vi "UHR-Fleezers Control (host) - 12.3.1.vi"() -> ()   [LabVIEW 2012] (continued)
      tunnel: [_ _ _ _ _ _ _ _ _ w1722 _ _ _ _ _ _ _ _ _ _ _ _ _ _ _ _ _ _ _ _ _ _ _ _ _ _ _ _ _ _ _ _ _ _ _ _ _ _ _ _ _ _ _ _ _ _ _ _ _ _ _ _ _ _ _ _ _ _ _ _ _ _ _ _] -> w1588
      tunnel: [_ _ _ _ _ _ _ "Round T1 X" _ _ _ _ _ _ _ _ _ _ _ _ _ _ _ _ _ _ _ _ _ _ _ _ _ _ _ _ _ _ _ _ _ _ _ _ _ _ _ _ _ _ _ _ _ _ _ _ _ _ _ _ _ _ _ _ _ _ _ _ _ _ _ _ _ _] -> _
      tunnel: [_ _ _ "Adjust Scale\nto Mean" _ _ _ _ _ _ _ _ _ _ _ _ _ _ _ _ _ _ _ _ _ _ _ _ "Test ttrig" _ _ _ _ _ _ _ _ _ _ _ _ _ _ _ _ _ _ "Flush Sample" "Flush Pump 3" "Flush Pump 1" "Clear Volume" _ _ _ _ _ _ _ _ _ _ _ _ _ _ _ _ _ _ _ _ _ _ _] -> _
      tunnel: [_ _ _ _ _ _ _ _ "Round T2 X" _ "Delayed Interlace Start" _ _ _ _ _ _ _ _ _ _ _ _ _ _ _ _ _ _ _ _ _ _ _ _ _ _ _ _ _ _ _ _ _ _ _ _ _ _ _ _ _ _ _ _ _ _ _ _ _ _ _ _ _ _ _ _ _ _ _ _ _ _ _] -> _
      tunnel: w1587 -> [_ _ _ _ _ _ _ _ _ _ _ _ _ _ _ _ _ _ _ _ _ _ _ _ _ _ _ _ _ _ _ _ _ _ _ _ _ _ _ _ _ _ _ w2437 w2444 w2451 w2456 w2465 _ _ w2571 _ _ _ _ _ _ _ _ _ _ _ _ _ _ _ _ _ _ _ _ _ _ _]
      tunnel: w1586 -> [_ _ _ _ _ _ _ _ _ _ _ _ _ _ _ _ _ _ _ _ _ _ _ _ _ _ _ _ _ _ _ _ _ _ _ _ _ _ _ _ _ w2354 _ _ _ _ _ _ w2509 _ _ w2577 _ w2586 _ w2600 _ _ _ _ _ _ _ _ _ _ _ _ _ _ _ _ _ _]
      tunnel: w1585 -> [_ _ _ _ _ _ _ _ _ _ _ _ _ _ _ _ _ _ _ _ _ _ _ _ _ _ _ _ _ _ _ _ _ _ _ _ _ _ _ _ _ _ _ _ _ _ _ _ _ _ _ _ _ _ _ _ _ _ _ _ _ _ _ _ _ _ _ _ _ _ _ _ _ _]
      tunnel: w1584 -> [_ _ _ _ _ _ _ _ _ _ _ _ _ _ _ _ _ _ _ _ _ _ _ _ _ _ _ _ _ _ _ _ _ _ _ _ _ _ _ _ w2291 _ _ _ _ _ _ _ _ w2539 _ _ w2582 _ w2593 _ w2625 _ _ _ _ _ _ _ _ _ _ _ _ _ _ _ _ _]
      tunnel: w1583 -> [_ _ _ _ _ _ _ _ _ _ _ _ _ _ _ _ _ _ _ _ _ _ _ _ _ _ _ _ _ _ _ _ _ _ _ _ _ _ _ _ _ _ _ _ _ _ _ _ _ _ _ _ _ _ _ _ _ _ _ _ _ _ _ _ _ _ _ _ _ _ _ _ _ _]
      event "AI Count (ticks)", "Sets to FIFO (Traps)", "Save ave N", "FPGA Ave.", "# Samples/channel", "N sets to save": Value Change {
        # "So that if 'Save ave N' is updated, the AOD scanning code updates too."
        n1098 = event-data() -> ()  [unwired: 6 out]
        n1099 = local read "AI Count (ticks)"() -> (w1614:u16)
        n1100 = Unbundle By Name("Sets to FIFO (Traps)") -> ("Set 1"=w1597:bool, "Set 2"=w1596:bool, "Set 3"=w1595:bool)
        n1101 = Boolean To (0,1)(Boolean="Sets to FIFO (Traps)") -> (0, 1=w1622:cluster{"Set 1":i16, "Set 2":i16, "Set 3":i16})
        n1102 = xnode "Read/Write Control"("FPGA VI Reference In"=w1632, "error in"=w1630, "ai count"=w1614, "Set 1"=w1597, "Set 2"=w1596, "Set 3"=w1595, "N of AI1 Int Acq Sets"="N Acq Sets (Traps + Fl.)") -> ("error out"=w1631:errorcluster)  [unwired: 1 out]
        n1103 = Cluster To Array(cluster=w1622) -> (array=w1621:i16[])
        n1104 = To Unsigned Long Integer(number=w1621) -> (unsigned 32bit integer=w1603:u32[])
        n1105 = local read "Scan steps (AOD)"() -> (w1623:u64)
        n1106 = Multiply(x=w1614, y="N Acq Sets (Traps + Fl.)") -> (x*y=w1612:u16)
        n1107 = Divide(x=40000000.0, y=w1614) -> (x/y=w1606:dbl)
        "AI rate (Hz)" <- w1606
        "Ave. Rate (Hz)" <- w1606
        n1108 = Add Array Elements(numeric array=w1603) -> (sum=w1615:u32)
        "Trap Sets" <- w1615
        n1109 = Reciprocal(x=w1606) -> (1/x=→"Ave. Period (s)":dbl)
        n1110 = property on="Scan steps (AOD)" class="DigNum (strict)"("Val(Sgnl)"=w1623) -> ()  [unwired: 2 in, 2 out]
        n1111 = Divide(x=w1606, y="N Acq Sets (Traps + Fl.)") -> (x/y=w1627:dbl)
        "Data Rate (Hz)" <- w1627
        n1112 = Reciprocal(x=w1627) -> (1/x=→"Data Period (s)":dbl)
        n1113 = local read "Save ave N"() -> (w1626:dbl)
        n1114 = Divide(x=w1627, y=w1626) -> (x/y=w1625:dbl)
        "Save Data Rate (Hz)" <- w1625
        n1115 = Reciprocal(x=w1625) -> (1/x=→"Save Data Period (s)":dbl)
        n1116 = Multiply(x=w1612, y="# Samples/trap") -> (x*y=w1610:u32)
        "Counts/DMA" <- w1610
        n1117 = property on="Trap Disp. Downsample" class="DigNum (strict)"("Maximum"="# Samples/trap") -> ()  [unwired: 2 in, 2 out]
        n1118 = Multiply(x=w1615, y="# Samples/trap") -> (x*y=w1604:u32)
        "# Samples/channel" <- w1604
        n1119 = Multiply(x=w1604, y=u32 8) -> (x*y=→"Trap AI Elements/DMA read":u32)
        n1120 = local read "APD Int. Count"() -> (w1611:u32)
        n1121 = Multiply(x=w1604, y=u32 3) -> (x*y=→"Trap Pos Elements/DMA read":u32)
        n1122 = Divide(x=w1610, y=w1611) -> (x/y=w1601:dbl)
        "APD Samples/FIFO Acq." <- w1601
        n1123 = Divide(x=w1610, y=40000000.0) -> (x/y=w1608:dbl)
        "DMA Update Period (s)" <- w1608
        n1124 = local read "Number of APDs"() -> (w1594:u8)
        n1125 = Multiply(x=w1594, y=w1601) -> (x*y=→"APD Elements/DMA read":dbl)
        n1126 = property on="APD Disp. Downsample" class="DigNum (strict)"("Maximum"=w1601) -> ()  [unwired: 2 in, 2 out]
        n1127 = local read "N sets to save"() -> (w1620:u32)
        n1128 = Multiply(x=w1608, y=w1620) -> (x*y=→"Total Time (s)":dbl)
        "FPGA Averaging" <- FALSE ("FPGA Averaging")
      }
      event "Remove Offset": Value Change {
        n1129 = event-data() -> ()  [unwired: 7 out]
        n1130 = local write "Remove Offset"(FALSE ("Remove Offset")) -> ()
        n1131 = local read "Bead Mean (nm)"() -> (w1634:dbl)
        n1132 = local read "Offset (nm)"() -> (w1635:dbl)
        n1133 = Add(x=w1634, y=w1635) -> (x+y=w1633:dbl)
        n1134 = local write "Offset (nm)"(w1633) -> ()
        n1135 = disable-structure shown="Disabled" {
          frame Disabled {
            n1136 = local read "Bead Mean (nm)"() -> (w1640:dbl)
            n1137 = Add(y=w1640) -> (x=w1639:dbl, x+y=w1638:dbl)
            n1138 = Subtract(x=w1640, y=w1639) -> (x-y=w1637:dbl)
            n1139 = property on="Bead Separation" class="WFChart (strict)"("YScale.Minimum"=w1637) -> ()  [unwired: 2 in, 2 out]
            n1140 = property on="Bead Separation" class="WFChart (strict)"("YScale.Maximum"=w1638) -> ()  [unwired: 2 in, 2 out]
          }
          frame Enabled {
          }
        }
      }
      event "Detector Type": Value Change {
        n1141 = event-data() -> ()  [unwired: 7 out]
        n1142 = local read "AI labels"() -> (w1641:string[])
        n1143 = property on="High Res. Display" class="Ring (strict)"("Strings []"=w1641) -> ()  [unwired: 2 in, 2 out]
        n1144 = Build Array (concatenate)(w1641, "none") -> (w1642:string[])
        n1145 = property on="FFT 1 Choice 1" class="Ring (strict)"("Strings []"=w1642) -> ()  [unwired: 2 in, 2 out]
        n1146 = property on="FFT 1 Choice 2" class="Ring (strict)"("Strings []"=w1642) -> ()  [unwired: 2 in, 2 out]
        n1147 = property on="FFT 2 Choice 1" class="Ring (strict)"("Strings []"=w1642) -> ()  [unwired: 2 in, 2 out]
        n1148 = property on="FFT 2 Choice 2" class="Ring (strict)"("Strings []"=w1642) -> ()  [unwired: 2 in, 2 out]
        n1149 = Bundle("APD 1", "APD 2") -> (w1645:cluster{string, string})  [unwired: 1 out]
        n1150 = Cluster To Array(cluster=w1645) -> (array=w1643:string[])
        n1151 = Build Array (concatenate)(w1643, w1642) -> (w1647:string[])
        n1152 = Array Size(array=w1647) -> (size(s)=w1648:i32)
        n1153 = property on="Signals to Plot" class="LstBox (strict)"("Item Names"=w1647) -> ()  [unwired: 2 in, 2 out]
        n1154 = property on="Signals to Plot" class="LstBox (strict)"("Number of Rows"=w1648) -> ()  [unwired: 2 in, 2 out]
        n1155 = property on="All Signals" class="WFChart (strict)"("LegNumRows"=w1648) -> ()  [unwired: 2 in, 2 out]
      }
      event "Adjust Scale\nto Mean": Value Change {
        n1156 = event-data() -> ()  [unwired: 7 out]
        n1157 = local read "APD 1 Rate (Hz)"() -> (w1657:dbl)
        n1158 = Multiply(x=1000.0, y="Above (kHz)") -> (x*y=w1655:dbl)
        n1159 = Multiply(x=1000.0, y="Below (kHz)") -> (x*y=w1653:dbl)
        n1160 = Add(x=w1655, y=w1657) -> (x+y=w1650:dbl)
        n1161 = Subtract(x=w1657, y=w1653) -> (x-y=w1651:dbl)
        n1162 = property on="APD Chart" class="WFChart (strict)"("YScale.Minimum"=w1651) -> ()  [unwired: 2 in, 2 out]
        n1163 = property on="APD Chart" class="WFChart (strict)"("YScale.Maximum"=w1650) -> ()  [unwired: 2 in, 2 out]
      }
      event "Phase adj. (AI1)", "+ phase (AI1)", "- phase (AI1)": Value Change {
        n1164 = event-data() -> ()  [unwired: 7 out]
        n1165 = Negate(x="Phase adj. (AI1)") -> (-x=w1667:i16)
        n1166 = Select(t=w1667, s="- phase (AI1)", f="Phase adj. (AI1)") -> (s? t:f=w1666:i16)
        n1167 = xnode "Read/Write Control"("FPGA VI Reference In"=w1670, "error in"=w1669, "Phase count adjustment"=w1666) -> ("FPGA VI Reference Out"=w1665:T19, "error out"=w1664:errorcluster)
        n1168 = Or(x="- phase (AI1)", y="+ phase (AI1)") -> (x .or. y?=w1661:bool)
        n1169 = xnode "Read/Write Control"("FPGA VI Reference In"=w1665, "error in"=w1664, "+ phase"=w1661) -> ("error out"=w1660:errorcluster)  [unwired: 1 out]
      }
      event "Signals to Plot": Double Click {
        w1673 = u32 9868950 ("Color Box")
        n1170 = event-data() -> ("Row"=w1675:i32)  [unwired: 9 out]
        n1171 = property on="All Signals" class="WFChart (strict)"("Active Plot"=w1675) -> (error out=w1686:errorcluster)  [unwired: 2 in, 1 out]
        n1172 = property on="All Signals" class="WFChart (strict)" props=["Plot", "Visible?", "Plot", "Plot Color"](error in=w1686) -> (error out=w1685:errorcluster, "Plot.Visible?"=w1684:bool)  [unwired: 1 in, 2 out]
        n1173 = Select(t=FALSE ("Plot.Visible"), s=w1684, f=TRUE ("Plot.Visible")) -> (s? t:f=w1679:bool)
        n1174 = property on="All Signals" class="WFChart (strict)"(error in=w1685, "Plot.Visible?"=w1679) -> (error out=w1681:errorcluster)  [unwired: 1 in, 1 out]
        n1175 = property on="All Signals" class="WFChart (strict)"(error in=w1681) -> (error out=w1676:errorcluster, "Plot.Plot Color"=w1680:u32)  [unwired: 1 in, 1 out]
        n1176 = property on="Signals to Plot" class="LstBox (strict)"(error in=w1676, "Active Row"=w1675) -> (error out=w1674:errorcluster)  [unwired: 1 in, 1 out]
        n1177 = Select(t=w1680, s=w1679, f=u32 0) -> (s? t:f=w1677:u32)
        n1178 = property on="Signals to Plot" class="LstBox (strict)"(error in=w1674, "CellFontColor"=w1677, "SelColor"=w1673, "CellBG"=w1673, "CellFontSize"=u32 20 ("Active Row:Cell Font:Size"), "CellFontBold"=TRUE ("Active Row:Cell Font:Bold")) -> ()  [unwired: 1 in, 2 out]
      }
      event "BD 1 Frequency 1 (MHz)", "BD 1 Frequency 2 (MHz)", "BD 1 Frequency 3 (MHz)", "BD 2 Frequency 1 (MHz)", "BD 2 Frequency 2 (MHz)", "BD 2 Frequency 3 (MHz)", "Trap Delta (MHz)": Value Change {
        n1179 = event-data() -> ("CtlRef"=w1689:refnum<vi>)  [unwired: 6 out]
        n1180 = control-ref of="Trap Delta (MHz)"() -> (w1688:refnum<vi>)
        n1181 = Equal?(x=w1688, y=w1689) -> (x = y?=w1687:bool)
        n1182 = case shown="False" "Oscillate Set 1" {
          tunnel: w1692 -> [w1712 _]
          tunnel: [w1711 w1715] -> w1691
          tunnel: w1690 -> [w1710 w1715]
          tunnel: w1687 -> [w1695 _]
          frame False {
            n1183 = local read "BD 1 Frequency 2 (MHz)"() -> (w1699:dbl)
            n1184 = local read "BD 1 Frequency 1 (MHz)"() -> (w1697:dbl)
            n1185 = Subtract(x=w1699, y="Trap Delta (MHz)") -> (x-y=w1696:dbl)
            n1186 = Select(t=w1696, s=w1695, f=w1697) -> (s? t:f=w1694:dbl)
            n1187 = local read "Y RF Frequency Limits (MHz)"() -> (w1700:T16)
            n1188 = local read "X RF Frequency Limits (MHz)"() -> (w1701:T16)
            n1189 = local read "BD 1 Frequency 3 (MHz)"() -> (w1713:dbl)
            n1190 = local write "BD 1 Frequency 1 (MHz)"(w1694) -> ()
            n1191 = local read "BD 2 Frequency 1 (MHz)"() -> (w1704:dbl)
            n1192 = local read "BD 2 Frequency 2 (MHz)"() -> (w1703:dbl)
            n1193 = local read "BD 2 Frequency 3 (MHz)"() -> (w1714:dbl)
            n1194 = call "set RF board frequency - interlace.vi"("Board 2 Frequency Limits"=w1700, "Board 1 Frequency Limits"=w1701, "error in"=w1710, "FPGA VI Reference In"=w1712, "Board 2 Frequency 3 (MHz)"=w1714, "Board 1 Frequency 3 (MHz)"=w1713, "Board 2 Frequency 2 (MHz)"=w1703, "Board 2 Frequency 1 (MHz)"=w1704, "Board 1 Frequency 2 (MHz)"=w1699, "Board 1 Frequency 1  (MHz)"=w1694) -> ("error out"=w1711:errorcluster)  [unwired: 1 out]
            n1195 = Subtract(x=w1704, y=w1703) -> (x-y=w1708:dbl)
            n1196 = Subtract(x=w1694, y=w1699) -> (x-y=w1709:dbl)
            n1197 = Square(x=w1708) -> (x^2=w1706:dbl)
            n1198 = Square(x=w1709) -> (x^2=w1707:dbl)
            n1199 = Add(x=w1707, y=w1706) -> (x+y=w1705:dbl)
            n1200 = Square Root(x=w1705) -> (sqrt(x)=w1702:dbl)
            n1201 = local write "Trap Delta (MHz)"(w1702) -> ()
            n1202 = property on="Initial delta (MHz)" class="DigNum (strict)"("Val(Sgnl)"=w1702) -> ()  [unwired: 2 in, 2 out]
          }
          frame True {
          }
        }
      }
      event "Round T1 X": Value Change {
        n1203 = event-data() -> ()  [unwired: 7 out]
        n1204 = local read "BD 1 Frequency 1 (MHz)"() -> (w1718:dbl)
        n1205 = Round To Nearest(number=w1718) -> (nearest integer value=w1717:dbl)
        n1206 = property on="BD 1 Frequency 1 (MHz)" class="DigNum (strict)"("Val(Sgnl)"=w1717) -> ()  [unwired: 2 in, 2 out]
      }
      event "Round T2 X": Value Change {
        n1207 = event-data() -> ()  [unwired: 7 out]
        n1208 = local read "BD 1 Frequency 2 (MHz)"() -> (w1720:dbl)
        n1209 = Round To Nearest(number=w1720) -> (nearest integer value=w1719:dbl)
        n1210 = property on="BD 1 Frequency 2 (MHz)" class="DigNum (strict)"("Val(Sgnl)"=w1719) -> ()  [unwired: 2 in, 2 out]
      }
      event "Stop All": Value Change {
        n1211 = event-data() -> ()  [unwired: 7 out]
        n1212 = local read "Stop All"() -> (w1722:bool)
      }
      event "Delayed Interlace Start": Value Change {
        n1213 = event-data() -> ()  [unwired: 7 out]
        n1214 = flat-sequence {
          frame #0 {
            n1215 = Multiply(x="Delay to Interlace (s)", y=1000.0) -> (x*y=w1725:dbl)
            n1216 = Wait (ms)(milliseconds to wait=w1725) -> ()  [unwired: 1 out]
          }
          frame #1 {
            n1217 = property on="Laser interlacing mode" class="RadioBtnsControl (strict)"("Val(Sgnl)"=enum32{"Laser ON", "Laser OFF", "Interlace"}."Interlace" ("Value (Signaling)")) -> ()  [unwired: 2 in, 2 out]
          }
        }
      }
      event "BD 1 Amplitude 1 (%)", "BD 1 Amplitude 2 (%)", "BD 1 Amplitude 3 (%)", "BD 2 Amplitude 1 (%)", "BD 2 Amplitude 2 (%)", "BD 2 Amplitude 3 (%)", "Trap 1 ON", "Trap 2 ON", "Trap 3 ON", "Feedback On/Off", "All FB On/Off": Value Change {
        w1749 = i16 1 ("f")
        n1218 = event-data() -> ()  [unwired: 7 out]
        n1219 = local write "Trap 1 (ON/OFF)"("Trap 1 ON") -> ()
        n1220 = local write "Trap 2 (ON/OFF)"("Trap 2 ON") -> ()
        n1221 = Boolean To (0,1)(Boolean="Trap 3 ON") -> (0, 1=w1750:i16)
        n1222 = Boolean To (0,1)(Boolean="Trap 1 ON") -> (0, 1=w1751:i16)
        n1223 = Boolean To (0,1)(Boolean="Trap 2 ON") -> (0, 1=w1752:i16)
        n1224 = Select(t=w1752, s="Trap ON/OFF X or Y Amp?", f=w1749) -> (s? t:f=w1747:i16)
        n1225 = Select(t=w1751, s="Trap ON/OFF X or Y Amp?", f=w1749) -> (s? t:f=w1748:i16)
        n1226 = Select(t=w1750, s="Trap ON/OFF X or Y Amp?", f=w1749) -> (s? t:f=w1746:i16)
        n1227 = Select(t=w1749, s="Trap ON/OFF X or Y Amp?", f=w1752) -> (s? t:f=w1744:i16)
        n1228 = Select(t=w1749, s="Trap ON/OFF X or Y Amp?", f=w1751) -> (s? t:f=w1745:i16)
        n1229 = Select(t=w1749, s="Trap ON/OFF X or Y Amp?", f=w1750) -> (s? t:f=w1743:i16)
        n1230 = And(x="All FB On/Off", y="Feedback On/Off") -> (x .and. y?=w1741:cluster{"Set 1":bool, "Set 2":bool})
        n1231 = local read "BD 1 Amplitude 1 (%)"() -> (w1761:dbl)
        n1232 = local read "BD 1 Amplitude 2 (%)"() -> (w1760:dbl)
        n1233 = local read "BD 1 Amplitude 3 (%)"() -> (w1759:dbl)
        n1234 = Unbundle By Name(w1741) -> ("Set 1"=w1736:bool, "Set 2"=w1733:bool)
        n1235 = local read "Y RF Amplitude Limits (%)"() -> (w1729:T16)
        n1236 = local read "X RF Amplitude Limits (%)"() -> (w1730:T16)
        n1237 = local read "BD 2 Amplitude 1 (%)"() -> (w1762:dbl)
        n1238 = local read "BD 2 Amplitude 2 (%)"() -> (w1763:dbl)
        n1239 = local read "BD 2 Amplitude 3 (%)"() -> (w1764:dbl)
        n1240 = And(x="Trap 2 ON", y=w1733) -> (x .and. y?=w1731:bool)
        n1241 = And(x="Trap 1 ON", y=w1736) -> (x .and. y?=w1734:bool)
        n1242 = Multiply(x=w1748, y=w1761) -> (x*y=w1756:dbl)
        n1243 = Multiply(x=w1760, y=w1747) -> (x*y=w1754:dbl)
        n1244 = Multiply(x=w1759, y=w1746) -> (x*y=w1755:dbl)
        n1245 = Multiply(x=w1762, y=w1745) -> (x*y=w1765:dbl)
        n1246 = Multiply(x=w1763, y=w1744) -> (x*y=w1766:dbl)
        n1247 = Multiply(x=w1764, y=w1743) -> (x*y=w1767:dbl)
        n1248 = call "set RF board amplitude - interlace.vi"("Board 2 Amplitude Limits"=w1729, "Board 1 Amplitude Limits"=w1730, "error in"=w1757, "FPGA VI Reference In"=w1758, "Board 2 Amplitude 3 (%)"=w1767, "Board 1 Amplitude 3 (%)"=w1755, "Board 2 Amplitude 2 (%)"=w1766, "Board 2 Amplitude 1 (%)"=w1765, "Board 1 Amplitude 2 (%)"=w1754, "Board 1 Amplitude 1 (%)"=w1756) -> ("error out"=w1738:errorcluster, "FPGA VI Reference Out"=w1739:T19)
        n1249 = xnode "Read/Write Control"("FPGA VI Reference In"=w1739, "error in"=w1738, "FB On/Off Set 1"=w1734, "FB On/Off Set 2"=w1731) -> ("error out"=w1737:errorcluster)  [unwired: 1 out]
      }
      event "Load parameters": Value Change {
        n1250 = event-data() -> ()  [unwired: 7 out]
        n1251 = property on="Saved AOD Raster Scan Parameter Sets" class="Arr (strict)"() -> ("Index Values"=w1778:u32[])  [unwired: 2 in, 2 out]
        n1252 = Index Array(array=w1778, index=0) -> (element=w1775:u32)
        n1253 = local write "Load parameters"(FALSE ("Load parameters")) -> ()
        n1254 = Index Array(array="Saved AOD Raster Scan Parameter Sets", index=w1775) -> (element=w1774:T27)
        n1255 = Unbundle By Name(w1774) -> ("Scan Range AOD (nm) 2"=w1773:dbl, "Step Size AOD (nm) 2"=w1772:dbl, "Scan Speed AOD (nm/s) 2"=w1771:dbl, "Number of scans (AOD) 2"=w1770:u16)
        n1256 = flat-sequence {
          tunnel: w1773 -> [w1781]
          tunnel: w1772 -> [w1780]
          tunnel: w1771 -> [w1779]
          tunnel: w1770 -> [w1782]
          frame #0 {
            n1257 = local write "Scan Speed (nm/s)"(w1779) -> ()
            n1258 = local write "Scan Range (nm)"(w1781) -> ()
            n1259 = local write "Step Size (nm)"(w1780) -> ()
          }
          frame #1 {
            n1260 = property on="Number of F/B Scans (AOD)" class="DigNum (strict)"("Val(Sgnl)"=w1782) -> ()  [unwired: 2 in, 2 out]
          }
        }
      }
      event "Trap 1 (ON/OFF)", "Trap 2 (ON/OFF)": Value Change {
        n1261 = event-data() -> ()  [unwired: 7 out]
        n1262 = property on="Trap 2 ON" class="Bool (strict)"("Val(Sgnl)"="Trap 2 (ON/OFF)") -> ()  [unwired: 2 in, 2 out]
        n1263 = property on="Trap 1 ON" class="Bool (strict)"("Val(Sgnl)"="Trap 1 (ON/OFF)") -> ()  [unwired: 2 in, 2 out]
      }
      event "DIO count 1 (ticks)", "DIO count 2 (ticks)", "DIO count 3 (ticks)", "Interlace", "Number Interlace Sets", "Not-Interlacing Set": Value Change {
        n1264 = event-data() -> ()  [unwired: 7 out]
        n1265 = local read "DIO count 3 (ticks)"() -> (w1795:u16)
        n1266 = local read "DIO count 1 (ticks)"() -> (w1797:u16)
        n1267 = local read "DIO count 2 (ticks)"() -> (w1796:u16)
        n1268 = To Unsigned Byte Integer(number="Not-Interlacing Set") -> (unsigned 8bit integer=w1786:u8)
        n1269 = Add(x=w1786, y=u8 1) -> (x+y=w1790:u8)
        n1270 = xnode "Read/Write Control"("FPGA VI Reference In"=w1801, "error in"=w1799, "DIO count 1 (ticks)"=w1797, "DIO count 2 (ticks)"=w1796, "DIO count 3 (ticks)"=w1795, "Interlace ON/OFF"="Interlace", "Number Interlace Cycles"="Number Interlace Sets", "Interlace Off Parameters"=w1790) -> ("error out"=w1800:errorcluster)  [unwired: 1 out]
        n1271 = Build Array(w1797, w1796, w1795) -> (w1788:u16[])
        n1272 = Split 1D Array(array=w1788, index="Number Interlace Sets") -> (first subarray=w1798:u16[])  [unwired: 1 out]
        n1273 = Index Array(array=w1788, index=w1786) -> (element=w1787:u16)
        n1274 = Add Array Elements(numeric array=w1798) -> (sum=w1792:u16)
        n1275 = Select(t=w1792, s="Interlace", f=w1787) -> (s? t:f=→"Total Counts (ticks)":u16)
      }
      event "Reset Feedback": Value Change {
        n1276 = event-data() -> ()  [unwired: 7 out]
        n1277 = Unbundle By Name("Reset Feedback") -> ("Set 1"=w1805:bool, "Set 2"=w1804:bool)
        n1278 = xnode "Read/Write Control"("FPGA VI Reference In"=w1807, "error in"=w1802, "FB Reset Set 1"=w1805, "FB Reset Set 2"=w1804) -> ("error out"=w1803:errorcluster)  [unwired: 1 out]
      }
      event "Trap Intensity PID Gains": Value Change {
        n1279 = event-data() -> ()  [unwired: 7 out]
        n1280 = Unbundle By Name("Trap Intensity PID Gains") -> ("proportional gain (Kc)"=w1810:i16, "integral gain (Kc*Ts/Ti)"=w1809:i16, "derivative gain (Kc*Td/Ts)"=w1808:i16)
        n1281 = xnode "Read/Write Control"("FPGA VI Reference In"=w1814, "error in"=w1812, "P1"=w1810, "I1"=w1809, "D1"=w1808) -> ("error out"=w1813:errorcluster)  [unwired: 1 out]
      }
      event "AI2 to Setpoint", "Setpoints (V)": Value Change {
        n1282 = event-data() -> ()  [unwired: 7 out]
        n1283 = xnode "Read/Write Control"("FPGA VI Reference In"=w1819, "error in"=w1815) -> ("FPGA VI Reference Out"=w1818:T19, "error out"=w1817:errorcluster, "AI2 Y Sum Set 1"=w1826:i16, "AI2 Y Sum Set 2"=w1825:i16)
        n1284 = Cluster To Array(cluster="AI2 to Setpoint") -> (array=w1829:bool[])
        n1285 = local read "AI2 (V)"() -> (w1827:cluster{"Set 1":dbl, "Set 2":dbl})
        n1286 = Or Array Elements(Boolean array=w1829) -> (logical OR=w1830:bool)
        n1287 = Bundle By Name(cluster=w1827, "Set 1"=w1826, "Set 2"=w1825) -> (w1824:cluster{"Set 1":dbl, "Set 2":dbl})
        n1288 = Divide(x=w1824, y=3276.7) -> (x/y=w1823:cluster{"Set 1":dbl, "Set 2":dbl})
        "AI2 (V)" <- w1823
        n1289 = case shown="True" w1830 {
          tunnel: [w1833 w1850] -> w1822
          tunnel: "AI2 to Setpoint" -> [_ w1846]
          tunnel: "Setpoints (V)" -> [w1834 w1849]
          tunnel: w1823 -> [_ w1843]
          frame False {
            n1290 = Multiply(x=3276.7, y=w1834) -> (x*y=w1835:cluster{"Set 1":dbl, "Set 2":dbl})
            n1291 = To Word Integer(number=w1835) -> (16bit integer=w1833:cluster{"Set 1":i16, "Set 2":i16})
          }
          frame True {
            n1292 = Unbundle By Name(w1843) -> ("Set 1"=w1842:dbl, "Set 2"=w1841:dbl)
            n1293 = Unbundle By Name(w1849) -> ("Set 1"=w1848:dbl, "Set 2"=w1847:dbl)
            n1294 = Unbundle By Name(w1846) -> ("Set 1"=w1845:bool, "Set 2"=w1844:bool)
            n1295 = Select(t=w1842, s=w1845, f=w1848) -> (s? t:f=w1840:dbl)
            n1296 = Select(t=w1841, s=w1844, f=w1847) -> (s? t:f=w1839:dbl)
            n1297 = Bundle By Name(cluster=w1849, "Set 1"=w1840, "Set 2"=w1839) -> (w1837:cluster{"Set 1":dbl, "Set 2":dbl})
            n1298 = local write "Setpoints (V)"(w1837) -> ()
            n1299 = Multiply(x=3276.7, y=w1837) -> (x*y=w1838:cluster{"Set 1":dbl, "Set 2":dbl})
            n1300 = To Word Integer(number=w1838) -> (16bit integer=w1850:cluster{"Set 1":i16, "Set 2":i16})
          }
        }
        n1301 = Unbundle By Name(w1822) -> ("Set 1"=w1821:i16, "Set 2"=w1820:i16)
        n1302 = xnode "Read/Write Control"("FPGA VI Reference In"=w1818, "error in"=w1817, "FB Setpoint Set 1"=w1821, "FB Setpoint Set 2"=w1820) -> ("error out"=w1816:errorcluster)  [unwired: 1 out]
      }
      event "+ phase (GI)", "- phase (GI)", "+ phase (GI) 2", "- phase (GI) 2", "+ phase (RI)", "- phase (RI)", "+ phase (RI) 2", "- phase (RI) 2", "+ phase (Green FB)", "- phase (Green FB)", "+ phase (RI FB)", "- phase (RI FB)": Value Change {
        n1303 = event-data() -> ()  [unwired: 7 out]
        n1304 = Or(x="+ phase (GI)", y="- phase (GI)") -> (x .or. y?=w1903:bool)
        n1305 = Negate(x="Phase adj. (GI)") -> (-x=w1908:i16)
        n1306 = Select(t=w1908, s="+ phase (GI)", f="Phase adj. (GI)") -> (s? t:f=w1907:i16)
        n1307 = Or(x="+ phase (GI) 2", y="- phase (GI) 2") -> (x .or. y?=w1894:bool)
        n1308 = Negate(x="Phase adj. (GI) 2") -> (-x=w1899:i16)
        n1309 = Select(t=w1899, s="+ phase (GI) 2", f="Phase adj. (GI) 2") -> (s? t:f=w1895:i16)
        n1310 = Negate(x="Phase adj. (RI)") -> (-x=w1893:i16)
        n1311 = Or(x="+ phase (RI)", y="- phase (RI)") -> (x .or. y?=w1889:bool)
        n1312 = Select(t=w1893, s="+ phase (RI)", f="Phase adj. (RI)") -> (s? t:f=w1888:i16)
        n1313 = Negate(x="Phase adj. (RI) 2") -> (-x=w1887:i16)
        n1314 = Or(x="+ phase (RI) 2", y="- phase (RI) 2") -> (x .or. y?=w1876:bool)
        n1315 = Select(t=w1887, s="+ phase (RI) 2", f="Phase adj. (RI) 2") -> (s? t:f=w1883:i16)
        n1316 = Or(x="+ phase (Green FB)", y="- phase (Green FB)") -> (x .or. y?=w1877:bool)
        n1317 = Negate(x="Phase adj. (Green FB)") -> (-x=w1882:i16)
        n1318 = Select(t=w1882, s="+ phase (Green FB)", f="Phase adj. (Green FB)") -> (s? t:f=w1878:i16)
        n1319 = Or(x="+ phase (RI FB)", y="- phase (RI FB)") -> (x .or. y?=w1870:bool)
        n1320 = Negate(x="Phase adj. (RI FB)") -> (-x=w1875:i16)
        n1321 = Select(t=w1875, s="+ phase (RI FB)", f="Phase adj. (RI FB)") -> (s? t:f=w1871:i16)
        n1322 = Negate(x="Phase adj. (BI AO)") -> (-x=w1869:i16)
        n1323 = Or(x="+ phase (BI AO)", y="- phase (BI AO)") -> (x .or. y?=w1854:bool)
        n1324 = Select(t=w1869, s="+ phase (BI AO)", f="Phase adj. (BI AO)") -> (s? t:f=w1857:i16)
        n1325 = Negate(x="Phase adj. (BI DO)") -> (-x=w1865:i16)
        n1326 = Or(x="+ phase (BI DO)", y="- phase (BI DO)") -> (x .or. y?=w1853:bool)
        n1327 = Select(t=w1865, s="+ phase (BI DO)", f="Phase adj. (BI DO)") -> (s? t:f=w1856:i16)
        n1328 = Negate(x="Phase adj. (BI AI)") -> (-x=w1861:i16)
        n1329 = Or(x="+ phase (BI AI)", y="- phase (BI AI)") -> (x .or. y?=w1852:bool)
        n1330 = Select(t=w1861, s="+ phase (BI AI)", f="Phase adj. (BI AI)") -> (s? t:f=w1855:i16)
        n1331 = xnode "Read/Write Control"("FPGA VI Reference In"=w1910, "error in"=w1909, "Phase count adjustment (GI)"=w1907, "Phase count adjustment (GI) 2"=w1895, "Phase count adjustment (RI)"=w1888, "Phase count adjustment (RI) 2"=w1883, "Phase count adjustment (Green FB)"=w1878, "Phase count adjustment (Red FB)"=w1871, "Phase count adjustment (BI AO)"=w1857, "Phase count adjustment (BI D)"=w1856, "Phase count adjustment (Blue Int)"=w1855) -> ("FPGA VI Reference Out"=w1905:T19, "error out"=w1906:errorcluster)
        n1332 = xnode "Read/Write Control"("FPGA VI Reference In"=w1905, "error in"=w1906, "+ phase (GI)"=w1903, "+ phase (GI) 2"=w1894, "+ phase (RI)"=w1889, "+ phase (RI) 2"=w1876, "+ phase (Green FB)"=w1877, "+ phase (Red FB)"=w1870, "+ phase (BI AO)"=w1854, "+ phase (BI D)"=w1853, "+ phase (Blue Int)"=w1852) -> ("error out"=w1904:errorcluster)  [unwired: 1 out]
      }
      event "Green Laser ON/OFF", "Red Laser ON/OFF", "Blue Laser ON/OFF": Value Change {
        # "This loop shouldn't be initialized.  The main 'laser ON' settings should dominate and set the others."
        n1333 = event-data() -> ()  [unwired: 7 out]
        n1334 = property on="Red Laser ON" class="Bool (strict)"("Val(Sgnl)"="Red Laser ON/OFF") -> ()  [unwired: 2 in, 2 out]
        n1335 = property on="Blue Laser ON" class="Bool (strict)"("Val(Sgnl)"="Blue Laser ON/OFF") -> ()  [unwired: 2 in, 2 out]
        n1336 = property on="Green Laser ON" class="Bool (strict)"("Val(Sgnl)"="Green Laser ON/OFF") -> ()  [unwired: 2 in, 2 out]
      }
      event "Laser interlacing mode", "Green Laser ON", "Red Laser ON", "Blue Laser ON": Value Change {
        n1337 = event-data() -> ()  [unwired: 7 out]
        n1338 = local write "Green Laser ON/OFF"("Green Laser ON") -> ()
        n1339 = local write "Blue Laser ON/OFF"("Blue Laser ON") -> ()
        n1340 = local write "Red Laser ON/OFF"("Red Laser ON") -> ()
        n1341 = case shown="True" "Green Laser ON" {
          tunnel: "Laser interlacing mode" -> [_ w1947]
          tunnel: [enum32{"Laser ON", "Laser OFF", "Interlace"}."Laser OFF" ("Green laser mode") w1947] -> w1923
          tunnel: [FALSE w1943] -> w1922
          frame False {
          }
          frame True {
            n1342 = local read "Green FB On/Off"() -> (w1944:bool)
            n1343 = Equal?(x=w1947, y=enum32{"Laser ON", "Laser OFF", "Interlace"}."Interlace") -> (x = y?=w1945:bool)
            n1344 = And(x=w1945, y=w1944) -> (x .and. y?=w1943:bool)
          }
        }
        n1345 = case shown="True" "Red Laser ON" {
          tunnel: "Laser interlacing mode" -> [_ w1940]
          tunnel: [enum32{"Laser ON", "Laser OFF", "Interlace"}."Laser OFF" ("Green laser mode") w1940] -> w1919
          tunnel: [FALSE w1936] -> w1918
          frame False {
          }
          frame True {
            n1346 = local read "Red FB On/Off"() -> (w1937:bool)
            n1347 = Equal?(x=w1940, y=enum32{"Laser ON", "Laser OFF", "Interlace"}."Interlace") -> (x = y?=w1938:bool)
            n1348 = And(x=w1938, y=w1937) -> (x .and. y?=w1936:bool)
          }
        }
        n1349 = case shown="True" "Blue Laser ON" {
          tunnel: "Laser interlacing mode" -> [_ w1931]
          tunnel: [enum32{"Laser ON", "Laser OFF", "Interlace"}."Laser OFF" ("Green laser mode") w1931] -> w1915
          tunnel: [FALSE w1929] -> w1914
          frame False {
          }
          frame True {
            n1350 = local read "Blue FB On/Off"() -> (w1930:bool)
            n1351 = Equal?(x=w1931, y=enum32{"Laser ON", "Laser OFF", "Interlace"}."Interlace") -> (x = y?=w1932:bool)
            n1352 = And(x=w1932, y=w1930) -> (x .and. y?=w1929:bool)
          }
        }
        n1353 = xnode "Read/Write Control"("FPGA VI Reference In"=w1926, "error in"=w1924, "Operating Mode"=w1923, "Operating Mode 2"=w1923, "Green FB On/Off"=w1922, "Red Laser Operating Mode"=w1919, "RI Operating Mode 2"=w1919, "Red FB On/Off"=w1918, "BI Operating Mode (AO)"=w1915, "Blue Laser Operating Mode (D)"=w1915, "Blue FB On/Off"=w1914) -> ("error out"=w1925:errorcluster)  [unwired: 1 out]
      }
      event "Invert laser interlacing": Value Change {
        n1354 = event-data() -> ()  [unwired: 7 out]
        n1355 = xnode "Read/Write Control"("FPGA VI Reference In"=w1951, "error in"=w1949, "Invert GI"="Invert laser interlacing", "Invert GI 2"="Invert laser interlacing", "Invert RI"="Invert laser interlacing", "Invert RI 2"="Invert laser interlacing", "Invert BI (AO)"="Invert laser interlacing", "Invert BI (D)"="Invert laser interlacing") -> ("error out"=w1950:errorcluster)  [unwired: 1 out]
      }
      event "Green FB Setpoint (mV)", "Green FB Gains", "Green FB On/Off", "Green Intensity - FB OFF (%)", "Green int current ON count adj": Value Change {
        n1356 = event-data() -> ()  [unwired: 7 out]
        n1357 = local read "Green FB Setpoint (mV)"() -> (w1962:dbl)
        n1358 = Multiply(x=w1962, y=3.2767) -> (x*y=w1961:dbl)
        n1359 = local read "Green Intensity - FB OFF (%)"() -> (w1965:dbl)
        n1360 = Multiply(x=w1965, y=655.35) -> (x*y=w1966:dbl)
        n1361 = To Unsigned Word Integer(number=w1966) -> (unsigned 16bit integer=w1964:u16)
        n1362 = local read "Green int current ON count adj"() -> (w1968:u32)
        n1363 = local read "Laser interlacing mode"() -> (w1958:enum32{"Laser ON", "Laser OFF", "Interlace"})
        n1364 = local read "Green FB Gains"() -> (w1955:T9)
        n1365 = local read "Green Laser ON"() -> (w1959:bool)
        n1366 = local read "Green FB On/Off"() -> (w1969:bool)
        n1367 = Equal?(x=w1958, y=enum32{"Laser ON", "Laser OFF", "Interlace"}."Interlace") -> (x = y?=w1956:bool)
        n1368 = Unbundle By Name(w1955) -> ("proportional gain (Kc)"=w1954:i16, "integral gain (Kc*Ts/Ti)"=w1953:i16, "derivative gain (Kc*Td/Ts)"=w1952:i16)
        n1369 = Compound Arithmetic op=AND(w1956, w1969, w1959) -> (w1960:bool)
        n1370 = xnode "Read/Write Control"("FPGA VI Reference In"=w1972, "error in"=w1971, "Green FB Setpoint"=w1961, "Green FB On/Off"=w1960, "Current Out"=w1964, "Green int current ON count adj"=w1968, "P3"=w1954, "I3"=w1953, "D3"=w1952) -> ("error out"=w1970:errorcluster)  [unwired: 1 out]
      }
      event "Blue FB Setpoint (mV)", "Blue FB Gains", "Blue FB On/Off", "Blue Intensity - FB OFF (%)", "Blue int AO ON count adjust": Value Change {
        # "16 bit analog out"
        n1371 = event-data() -> ()  [unwired: 7 out]
        n1372 = Multiply(x="Blue FB Setpoint (mV)", y=3.2767) -> (x*y=w1986:dbl)
        n1373 = Multiply(x="Blue Intensity - FB OFF (%)", y=655.35) -> (x*y=w1989:dbl)
        n1374 = To Unsigned Word Integer(number=w1989) -> (unsigned 16bit integer=w1988:u16)
        n1375 = local read "Laser interlacing mode"() -> (w1984:enum32{"Laser ON", "Laser OFF", "Interlace"})
        n1376 = Unbundle By Name("Blue FB Gains") -> ("proportional gain (Kc)"=w1981:i16, "integral gain (Kc*Ts/Ti)"=w1980:i16, "derivative gain (Kc*Td/Ts)"=w1979:i16)
        n1377 = local read "Blue Laser ON"() -> (w1973:bool)
        n1378 = Equal?(x=w1984, y=enum32{"Laser ON", "Laser OFF", "Interlace"}."Interlace") -> (x = y?=w1982:bool)
        n1379 = Compound Arithmetic op=AND(w1982, "Blue FB On/Off", w1973) -> (w1985:bool)
        n1380 = xnode "Read/Write Control"("FPGA VI Reference In"=w1993, "error in"=w1992, "Blue FB Setpoint"=w1986, "Blue FB On/Off"=w1985, "BI Current Out"=w1988, "Blue current ON count adj (AO)"="Blue int AO ON count adjust", "P5"=w1981, "I5"=w1980, "D5"=w1979) -> ("error out"=w1991:errorcluster)  [unwired: 1 out]
      }
      event "Red FB Setpoint (mV)", "Red FB Gains", "Red FB On/Off", "Red Intensity - FB OFF (%)", "Red int current ON count adj": Value Change {
        n1381 = event-data() -> ()  [unwired: 7 out]
        n1382 = local read "Red FB Setpoint (mV)"() -> (w2005:dbl)
        n1383 = Multiply(x=w2005, y=3.2767) -> (x*y=w2004:dbl)
        n1384 = local read "Red Intensity - FB OFF (%)"() -> (w1994:dbl)
        n1385 = Multiply(x=w1994, y=655.35) -> (x*y=w2008:dbl)
        n1386 = To Unsigned Word Integer(number=w2008) -> (unsigned 16bit integer=w2007:u16)
        n1387 = local read "Red int current ON count adj"() -> (w2010:u16)
        n1388 = local read "Laser interlacing mode"() -> (w2001:enum32{"Laser ON", "Laser OFF", "Interlace"})
        n1389 = local read "Red FB Gains"() -> (w1998:T9)
        n1390 = local read "Red Laser ON"() -> (w2002:bool)
        n1391 = local read "Red FB On/Off"() -> (w2011:bool)
        n1392 = Equal?(x=w2001, y=enum32{"Laser ON", "Laser OFF", "Interlace"}."Interlace") -> (x = y?=w1999:bool)
        n1393 = Unbundle By Name(w1998) -> ("proportional gain (Kc)"=w1997:i16, "integral gain (Kc*Ts/Ti)"=w1996:i16, "derivative gain (Kc*Td/Ts)"=w1995:i16)
        n1394 = Compound Arithmetic op=AND(w1999, w2011, w2002) -> (w2003:bool)
        n1395 = xnode "Read/Write Control"("FPGA VI Reference In"=w2014, "error in"=w2013, "Red FB Setpoint"=w2004, "Red FB On/Off"=w2003, "RI Current Out"=w2007, "Red int current ON count adj"=w2010, "P4"=w1997, "I4"=w1996, "D4"=w1995) -> ("error out"=w2012:errorcluster)  [unwired: 1 out]
      }
      event "+ phase (APD 1 Gate)", "- phase (APD 1 Gate)", "+ phase (APD 2 Gate)", "- phase (APD 2 Gate)", "+ phase (APD 3 Gate)", "- phase (APD 3 Gate)", "+ phase (APD Acq)", "- phase (APD Acq)": Value Change {
        n1396 = event-data() -> ()  [unwired: 7 out]
        n1397 = local read "Phase Adj. (APD 1 Gate)"() -> (w2034:i16)
        n1398 = Or(x="- phase (APD 1 Gate)", y="+ phase (APD 1 Gate)") -> (x .or. y?=w2036:bool)
        n1399 = Negate(x=w2034) -> (-x=w2041:i16)
        n1400 = Select(t=w2041, s="+ phase (APD 1 Gate)", f=w2034) -> (s? t:f=w2040:i16)
        n1401 = local read "Phase Adj. (APD 2 Gate)"() -> (w2031:i16)
        n1402 = Or(x="- phase (APD 2 Gate)", y="+ phase (APD 2 Gate)") -> (x .or. y?=w2029:bool)
        n1403 = Negate(x=w2031) -> (-x=w2033:i16)
        n1404 = Select(t=w2033, s="+ phase (APD 2 Gate)", f=w2031) -> (s? t:f=w2030:i16)
        n1405 = Negate(x="Phase Adj. (APD 3 Gate)") -> (-x=w2028:i16)
        n1406 = Or(x="- phase (APD 3 Gate)", y="+ phase (APD 3 Gate)") -> (x .or. y?=w2024:bool)
        n1407 = Select(t=w2028, s="+ phase (APD 3 Gate)", f="Phase Adj. (APD 3 Gate)") -> (s? t:f=w2025:i16)
        n1408 = local read "Phase Adj. (APD Acq)"() -> (w2022:i16)
        n1409 = Or(x="- phase (APD Acq)", y="+ phase (APD Acq)") -> (x .or. y?=w2020:bool)
        n1410 = Negate(x=w2022) -> (-x=w2023:i16)
        n1411 = Select(t=w2023, s="+ phase (APD Acq)", f=w2022) -> (s? t:f=w2021:i16)
        n1412 = xnode "Read/Write Control"("FPGA VI Reference In"=w2043, "error in"=w2042, "Phase count adjustment (APD 1 Gate)"=w2040, "Phase count adjustment (APD 2 Gate)"=w2030, "Phase count adjustment (APD 3 Gate)"=w2025, "Phase Count Adjustment (APD Acq)"=w2021) -> ("FPGA VI Reference Out"=w2038:T19, "error out"=w2039:errorcluster)
        n1413 = xnode "Read/Write Control"("FPGA VI Reference In"=w2038, "error in"=w2039, "+ phase (APD 1 Gate)"=w2036, "+ phase (APD 2 Gate)"=w2029, "+ phase (APD 3 Gate)"=w2024, "+ phase (APD Acq)"=w2020) -> ("error out"=w2037:errorcluster)  [unwired: 1 out]
      }
      event "Invert APD Gate", "APD Gate ON Count", "APD Gate OFF Count", "APD Gate", "APD Integration Time (s)", "APD AO Scale Factor", "Duty Frequency (ON 1/N cycles)": Value Change {
        n1414 = event-data() -> ()  [unwired: 7 out]
        n1415 = Add(x="Interlace ON count", y="Interlace OFF count") -> (x+y=w2049:u16)
        n1416 = Add(x="APD Gate ON Count", y="APD Gate OFF Count") -> (x+y=w2060:u16)
        n1417 = Multiply(x="Duty Frequency (ON 1/N cycles)", y=w2049) -> (x*y=w2045:u16)
        "Green AI Count" <- w2045
        "Red AI Count" <- w2045
        "Blue AI Count" <- w2045
        n1418 = Subtract(x=w2045, y="Interlace ON count") -> (x-y=w2048:u16)
        n1419 = Multiply(x=w2060, y="Duty Frequency (ON 1/N cycles)") -> (x*y=w2059:u16)
        n1420 = Subtract(x=w2059, y="APD Gate ON Count") -> (x-y=w2058:u16)
        n1421 = local read "DMA Update Period (s)"() -> (w2061:dbl)
        n1422 = Multiply(x="APD Integration Time (s)", y=40000000.0) -> (x*y=w2065:dbl)
        n1423 = Reciprocal(x="APD Integration Time (s)") -> (1/x=→"APD Acq Rate (Hz)":dbl)
        n1424 = To Unsigned Long Integer(number=w2065) -> (unsigned 32bit integer=w2051:u32)
        "APD Int. Count" <- w2051
        n1425 = local read "Number of APDs"() -> (w2044:u8)
        n1426 = Divide(x=w2061, y="APD Integration Time (s)") -> (x/y=w2063:dbl)
        n1427 = Multiply(x=w2044, y=w2063) -> (x*y=w2062:dbl)
        n1428 = local write "APD Samples/FIFO Acq."(w2063) -> ()
        n1429 = local write "APD Elements/DMA read"(w2062) -> ()
        n1430 = xnode "Read/Write Control"("FPGA VI Reference In"=w2069, "error in"=w2068, "Invert APD Gate"="Invert APD Gate", "APD Gate ON Count"="APD Gate ON Count", "APD Gate OFF Count"=w2058, "APD Acq Rate Count"=w2051, "APD Gate Operating Mode"="APD Gate", "APD AO scale factor"="APD AO Scale Factor", "Green interlace ON count"="Interlace ON count", "Green interlace OFF count"=w2048, "Green interlace ON count 2"="Interlace ON count", "Green interlace OFF count 2"=w2048, "Green FB Count"=w2045, "Red interlace ON count"="Interlace ON count", "Red interlace OFF count"="Interlace OFF count", "Red FB Count"=w2045, "Red interlace ON count 2"="Interlace ON count", "Red interlace OFF count 2"="Interlace OFF count", "Blue ON count (AO)"="Interlace ON count", "Blue OFF count (AO)"="Interlace OFF count", "Blue interlace OFF count (D)"="Interlace OFF count", "Blue interlace ON count (D)"="Interlace ON count", "Blue Int Count"=w2045) -> ("error out"=w2067:errorcluster)  [unwired: 1 out]
      }
      event "Neg. TTrig FPGA": Value Change {
        n1431 = event-data() -> ()  [unwired: 7 out]
        n1432 = xnode "Read/Write Control"("FPGA VI Reference In"=w2072, "error in"=w2071, "TTrig Negate Pos"="Neg. TTrig FPGA") -> ()  [unwired: 2 out]
      }
      event "Test ttrig": Value Change {
        n1433 = event-data() -> ()  [unwired: 7 out]
        n1434 = xnode "Read/Write Control"("FPGA VI Reference In"=w2076, "error in"=w2075, "TTrig?"=TRUE) -> ("error out"=w2074:errorcluster)  [unwired: 1 out]
      }
      event "Number of F/B Scans (AOD)", "Scan Speed (nm/s)", "Scan BD", "Initial delta (MHz)", "Step Size (nm)", "Scan Range (nm)": Value Change {
        w2139 = 123.0  # AOM cal (nm/MHz)
        n1435 = event-data() -> ()  [unwired: 7 out]
        n1436 = local read "BD 1 Frequency 1 (MHz)"() -> (w2122:dbl)
        n1437 = local read "AOM X Cal (nm/MHz)"() -> (w2114:dbl)
        n1438 = local read "X RF Frequency Limits (MHz)"() -> (w2126:T16)
        n1439 = local read "Y RF Frequency Limits (MHz)"() -> (w2123:T16)
        n1440 = local read "BD 2 Frequency 1 (MHz)"() -> (w2128:dbl)
        n1441 = Negate(x="Scan Range (nm)") -> (-x=w2092:dbl)
        n1442 = Divide(x=w2092, y=w2114) -> (x/y=w2096:dbl)
        n1443 = Select(t=w2126, s="Scan BD", f=w2123) -> (s? t:f=w2125:T16)
        n1444 = Select(t=w2122, s="Scan BD", f=w2128) -> (s? t:f=w2127:dbl)
        n1445 = Unbundle By Name(w2125) -> ("Maximum"=w2134:dbl, "Minimum"=w2133:dbl)
        n1446 = Add(x=w2096, y=w2127) -> (x+y=w2131:dbl)
        n1447 = Divide(x=w2092, y="Step Size (nm)") -> (x/y=w2111:dbl)
        n1448 = Divide(x="Step Size (nm)", y=w2114) -> (x/y=w2120:dbl)
        n1449 = Absolute Value(x=w2111) -> (abs(x)=w2095:dbl)
        n1450 = Sign(1:w2092) -> (0:w2093:dbl)
        n1451 = In Range and Coerce(upper limit=w2134, x=w2131, lower limit=w2133) -> (coerced(x)=w2130:dbl, In Range?=w2132:bool)
        n1452 = To Unsigned Quad Integer(1:w2095) -> (0:w2110:u64)
        "Scan steps (AOD)" <- w2110
        n1453 = call "IR AOM freq to word.vi"("Frequency In (MHz)"=w2120) -> ("Frequency Word Out (double)"=w2117:dbl)
        n1454 = Multiply(x=w2093, y=w2117) -> (x*y=w2094:dbl)
        n1455 = Subtract(x=w2131, y=w2130) -> (x-y=w2129:dbl)
        n1456 = To Quad Integer(1:w2094) -> (0:w2116:i64)
        "Incr. int (AOD)" <- w2116
        n1457 = Subtract(x=w2096, y=w2129) -> (x-y=w2115:dbl)
        "Scan Range (MHz)" <- w2115
        n1458 = Select(t=w2096, s=w2132, f=w2115) -> (s? t:f=w2135:dbl)
        n1459 = Multiply(x=w2115, y=w2114) -> (x*y=w2113:dbl)
        n1460 = Decrement(x=w2110) -> (x-1=w2163:u64)
        n1461 = Negate(x=w2113) -> (-x=w2109:dbl)
        n1462 = local write "Scan Range (nm)"(w2109) -> ()
        n1463 = Divide(x=w2135, y=w2163) -> (x/y=w2119:dbl)
        "Scan Increment (MHz)" <- w2119
        n1464 = call "IR AOM freq to word.vi"("Frequency In (MHz)"=w2119) -> ("Frequency Word Out (double)"=w2118:dbl)
        n1465 = Divide(x="Step Size (nm)", y="Scan Speed (nm/s)") -> (x/y=w2106:dbl)
        n1466 = To Quad Integer(1:w2118) -> ()  [unwired: 1 out]
        n1467 = local read "Number Interlace Sets"() -> (w2090:u8)
        n1468 = local read "AI Count (ticks)"() -> (w2091:u16)
        n1469 = local read "Total Counts (ticks)"() -> (w2089:u16)
        n1470 = local read "# Samples/trap"() -> (w2121:u32)
        n1471 = Multiply(x=w2091, y=w2090) -> (x*y=w2088:u16)
        n1472 = Divide(x=w2089, y=w2088) -> (x/y=w2087:dbl)
        n1473 = Select(t=w2122, s="Scan BD", f=w2128) -> (s? t:f=w2160:dbl)
        "Initial freq. (MHz)" <- w2160
        n1474 = Add(x=w2135, y=w2160) -> (x+y=→"Final freq. (MHz)":dbl)
        n1475 = Divide(x=w2089, y=40000000.0) -> (x/y=w2105:dbl)
        n1476 = Divide(x=w2106, y=w2105) -> (x/y=w2104:dbl)
        n1477 = To Unsigned Quad Integer(1:w2104) -> (0:w2079:u64)
        n1478 = Quotient & Remainder(x=w2079, y=u64 2) -> (x-y*floor(x/y)=w2083:u64)  [unwired: 1 out]
        n1479 = Equal?(x=w2083, y=u64 0) -> (x = y?=w2081:bool)
        n1480 = Decrement(x=w2079) -> (x-1=w2080:u64)
        n1481 = Select(t=w2079, s=w2081, f=w2080) -> (s? t:f=w2078:u64)
        "Cycles/step (AOD)" <- w2078
        n1482 = xnode "Read/Write Control"("FPGA VI Reference In"=w2171, "error in"=w2170, "Scan steps"=w2110, "Number of scans"="Number of F/B Scans (AOD)", "Cycles per step"=w2078, "Scan freq.  increment"=w2116, "Scan BD"="Scan BD") -> ("error out"=w2169:errorcluster)  [unwired: 1 out]
        n1483 = Multiply(x=w2110, y=w2078) -> (x*y=w2164:u64)
        n1484 = Multiply(x=w2164, y=u64 2) -> (x*y=w2086:u64)
        n1485 = Multiply(x=w2087, y=w2086) -> (x*y=w2085:dbl)
        "Data points/scan (f/b)" <- w2085
        n1486 = Multiply(x=w2085, y="Number of F/B Scans (AOD)") -> (x*y=w2167:dbl)
        "Data points/scans" <- w2167
        n1487 = Divide(x=w2167, y=w2121) -> (x/y=→"N sets should be saved":dbl)
        n1488 = Multiply(x=w2164, y=w2105) -> (x*y=w2103:dbl)
        "Time/Scan (s) (AOD)" <- w2103
        n1489 = Select(t=w2135, s="Scan BD", f=0.0) -> (s? t:f=w2161:dbl)
        n1490 = Select(t=0.0, s="Scan BD", f=w2135) -> (s? t:f=w2157:dbl)
        n1491 = local read "BD 2 Frequency 2 (MHz)"() -> (w2153:dbl)
        n1492 = local read "BD 1 Frequency 2 (MHz)"() -> (w2156:dbl)
        n1493 = Add(x=w2157, y=w2128) -> (x+y=w2154:dbl)
        n1494 = Add(x=w2122, y=w2161) -> (x+y=w2155:dbl)
        n1495 = Multiply(x=w2103, y=2.0) -> (x*y=w2102:dbl)
        n1496 = Multiply(x=w2102, y="Number of F/B Scans (AOD)") -> (x*y=w2099:dbl)
        n1497 = Divide(x=w2099, y=60.0) -> (x/y=→"Time to Finish All (min)":dbl)
        n1498 = Add(x="Trap 2 Bead Size (nm)", y="Trap 1 Bead Size (nm)") -> (x+y=w2143:dbl)
        n1499 = Divide(x=w2143, y=2.0) -> (x/y=w2137:dbl)
        n1500 = local read "Initial delta (MHz)"() -> (w2140:dbl)
        n1501 = Subtract(x=w2154, y=w2153) -> (x-y=w2151:dbl)
        n1502 = Subtract(x=w2155, y=w2156) -> (x-y=w2152:dbl)
        n1503 = Square(x=w2151) -> (x^2=w2150:dbl)
        n1504 = Square(x=w2152) -> (x^2=w2149:dbl)
        n1505 = Add(x=w2149, y=w2150) -> (x+y=w2148:dbl)
        n1506 = Square Root(x=w2148) -> (sqrt(x)=w2147:dbl)
        "Final delta (MHz)" <- w2147
        n1507 = Multiply(x=w2139, y=w2147) -> (x*y=w2146:dbl)
        n1508 = Multiply(x=w2140, y=w2139) -> (x*y=w2138:dbl)
        n1509 = Subtract(x=w2138, y=w2137) -> (x-y=→"Initial sep (nm)":dbl)
        n1510 = Subtract(x=w2146, y=w2137) -> (x-y=→"Final sep (nm)":dbl)
      }
      event "Freq or Amp switch first", "Swap F1 and F2", "Freq switch delay", "Amp switch delay": Value Change {
        n1511 = event-data() -> ()  [unwired: 7 out]
        n1512 = local read "Amp switch delay"() -> (w2172:u16)
        n1513 = local read "Swap F1 and F2"() -> (w2173:bool)
        n1514 = xnode "Read/Write Control"("FPGA VI Reference In"=w2176, "error in"=w2175, "Swap F1 and F2"=w2173, "Amp switch delay"=w2172) -> ("error out"=w2174:errorcluster)  [unwired: 1 out]
      }
      event "Scan steps (MCL)", "Number of scans (MCL)", "Scan Range (V)\n(of steps)", "2D or 1D Scan", "N APD Samp/step", "Fast Scan Dir", "Continuous MCL Scanning", "Scan lines (y)": Value Change {
        w2178 = 32767.0 ("y")
        n1515 = event-data() -> ()  [unwired: 7 out]
        n1516 = Select(t="Scan lines (y)", s="2D or 1D Scan", f="Number of scans (MCL)") -> (s? t:f=w2183:u64)
        n1517 = Decrement(x="Scan steps (MCL)") -> (x-1=w2199:u64)
        n1518 = Divide(x="Scan Range (V)\n(of steps)", y=w2199) -> (x/y=w2198:dbl)
        "Desired Scan Incr (V)" <- w2198
        n1519 = local read "APD Integration Time (s)"() -> (w2191:dbl)
        n1520 = Multiply(x=w2198, y=w2178) -> (x*y=w2207:dbl)
        n1521 = Divide(x=w2207, y=10.0) -> (x/y=w2197:dbl)
        "Desired incr (int)" <- w2197
        n1522 = local read "Update Count (MCL)"() -> (w2203:u32)
        n1523 = Round Toward -Infinity(1:w2197) -> (0:w2206:dbl)
        n1524 = To Word Integer(number=w2206) -> (16bit integer=w2181:i16)
        "Actual Incr. int (MCL)" <- w2181
        n1525 = Multiply(x=w2191, y=40000000.0) -> (x*y=w2204:dbl)
        n1526 = Divide(x=w2204, y=w2203) -> (x/y=w2202:dbl)
        n1527 = Multiply(x=i16 10, y=w2181) -> (x*y=w2179:i16)
        n1528 = Multiply(x="N APD Samp/step", y=w2202) -> (x*y=w2201:dbl)
        "Cycles/step (MCL)" <- w2201
        n1529 = Divide(x=w2179, y=w2178) -> (x/y=→"Actual MCL Inc (V)":dbl)
        n1530 = Multiply(x="N APD Samp/step", y="Scan steps (MCL)") -> (x*y=w2193:dbl)
        n1531 = local read "APD Samples/FIFO Acq."() -> (w2190:dbl)
        n1532 = Multiply(x=w2193, y=u64 2) -> (x*y=w2192:dbl)
        "Data points/scan (f+b)" <- w2192
        n1533 = Multiply(x=w2192, y=w2183) -> (x*y=w2210:dbl)
        "Data points/scans (MCL)" <- w2210
        n1534 = Multiply(x=w2191, y=w2192) -> (x*y=w2184:dbl)
        "Time/f+b scan (s) (MCL)" <- w2184
        n1535 = Divide(x=w2210, y=w2190) -> (x/y=→"N sets should be saved (MCL)":dbl)
        n1536 = Multiply(x=w2184, y=w2183) -> (x*y=→"Total Time (s)":dbl)
        n1537 = Not(x="Fast Scan Dir") -> (.not. x?=w2188:bool)
        n1538 = xnode "Read/Write Control"("FPGA VI Reference In"=w2214, "error in"=w2213, "Scan steps (MCL)"="Scan steps (MCL)", "Number of scans (MCL)"=w2183, "Cycles per step (MCL)"=w2201, "Scan freq.  increment (MCL)"=w2181, "1D or 2D Scan?"="2D or 1D Scan", "MCL Scan Axis"=w2188, "Cont. Scan (MCL)"="Continuous MCL Scanning") -> ("error out"=w2212:errorcluster)  [unwired: 1 out]
      }
      event "Read Cal": Value Change {
        w2216 = 1000.0 ("y")
        n1539 = event-data() -> ()  [unwired: 7 out]
        n1540 = local read "Save file name"() -> (w2241:path)
        n1541 = local write "Read Cal"(FALSE ("Read Cal")) -> ()
        n1542 = Strip Path(path=w2241) -> (stripped path=w2240:path)  [unwired: 1 out]
        n1543 = Path To String(path=w2240) -> (string=w2239:string)
        n1544 = Concatenate Strings(w2239, "\\current.cal" ("string")) -> (w2237:string)
        n1545 = String To Path(string=w2237) -> (path=w2236:path)
        n1546 = Open/Create/Replace File(file path (use dialog)=w2236, operation (0:open)=T26."open", access (0:read/write)=enum16{"read/write", "read-only", "write-only"}."read-only") -> (refnum out=w2244:refnum<file>, error out=w2230:errorcluster)  [unwired: 1 in, 3 out]
        n1547 = Deny Access(4:w2230, 7:w2244) -> (0:w2229:errorcluster, 3:w2235:refnum<file>)  [unwired: 1 out]
        n1548 = Read from Binary File(5:0.0, 8:w2229, 9:T25."big-endian, network order" ("byte order (0:big-endian, network order)"), 10:-1 ("count (1)"), 11:w2235) -> (0:w2228:errorcluster, 2:w2226:dbl[], 3:w2231:refnum<file>)  [unwired: 2 out]
        n1549 = Array To Cluster(array=w2226) -> (cluster=w2225:T28)
        n1550 = Unbundle(w2225) -> ("[0]"=w2224:dbl, "[1]"=w2223:dbl, "[2]"=w2222:dbl, "[3]"=w2221:dbl, "[4]"=w2220:dbl, "[5]"=w2219:dbl)
        n1551 = Close File(refnum=w2231, error in=w2228) -> (error out=→"Read cal error":errorcluster)  [unwired: 1 out]
        n1552 = Multiply(x=w2219, y=w2216) -> (x*y=w2217:dbl)
        n1553 = local write "T2 kappa_x (pN/nm)"(w2221) -> ()
        n1554 = local write "T1 kappa_x (pN/nm)"(w2222) -> ()
        n1555 = local write "T1 alpha_x (nm/V)"(w2224) -> ()
        n1556 = local write "T2 alpha_x (nm/V)"(w2223) -> ()
        n1557 = Multiply(x=w2220, y=w2216) -> (x*y=w2218:dbl)
        n1558 = local write "T1 offset_x (mV)"(w2218) -> ()
        n1559 = local write "T2 offset_x (mV)"(w2217) -> ()
      }
      event "Abort MCL Scan": Value Change {
        n1560 = event-data() -> ()  [unwired: 7 out]
        n1561 = local write "MCL Scanning"(FALSE ("MCL Scanning")) -> ()
        n1562 = xnode "Read/Write Control"("FPGA VI Reference In"=w2249, "error in"=w2248, "Abort scan (MCL)"="Abort MCL Scan") -> ("error out"=w2247:errorcluster)  [unwired: 1 out]
      }
      event "Update Count (MCL)": Value Change {
        n1563 = event-data() -> ()  [unwired: 7 out]
        n1564 = xnode "Read/Write Control"("FPGA VI Reference In"=w2253, "error in"=w2252, "MCL count"="Update Count (MCL)") -> ("error out"=w2251:errorcluster)  [unwired: 1 out]
      }
      event "+ phase (MCL)", "- phase (MCL)": Value Change {
        n1565 = event-data() -> ()  [unwired: 7 out]